vi "UHR-Fleezers Control (host) - 10.0.vi"() -> ()   [LabVIEW 2009] (continued)
  # "Harvard Pump\n(sample channel for flow exp)"
  # "Chemyx Pump 2"
  # "Units: \n1 = ml/m\n2 = ml/h\n3 = ul/m\n4 = ul/h"
  # "Rate param is ul/h\nVolume param is ul"
  # "X"
  # "Y"
  # "Oscillate Set 1 freq. (debugging)"
  # "BD 1"
  # "BD 2"
  # "AOD Raster Scan"
  # "Approx. trap separations"
  # "X"
  # "Y"
  # "APD Gates"
  # "APD 2"
  # "APD 1"
  # "X"
  # "2D"
  # "Y"
  # "1D"
  # "Green Laser Interlacing"
  # "Green FB Measurement"
  # "Digital Gate"
  # "Current Analog Control"
  # "Total AI Rates (NOT rates/trap)"
  # "(Samples/trap x Trap Sets)"
  # "(Samples/channel x\n8 if averaging (8 channels)\n4 if no averaging)"
  # "Trap 1"
  # "Trap 2"
  # "Flour./Trap 3"
  # "External Video Window"
  # "MCL Position Debugging"
  # "Temporary Control Storage\n(these used to be somewhere else, still want to keep them)"
  # "Y"
  # "X"
  # "Trap Position Difference Limits"
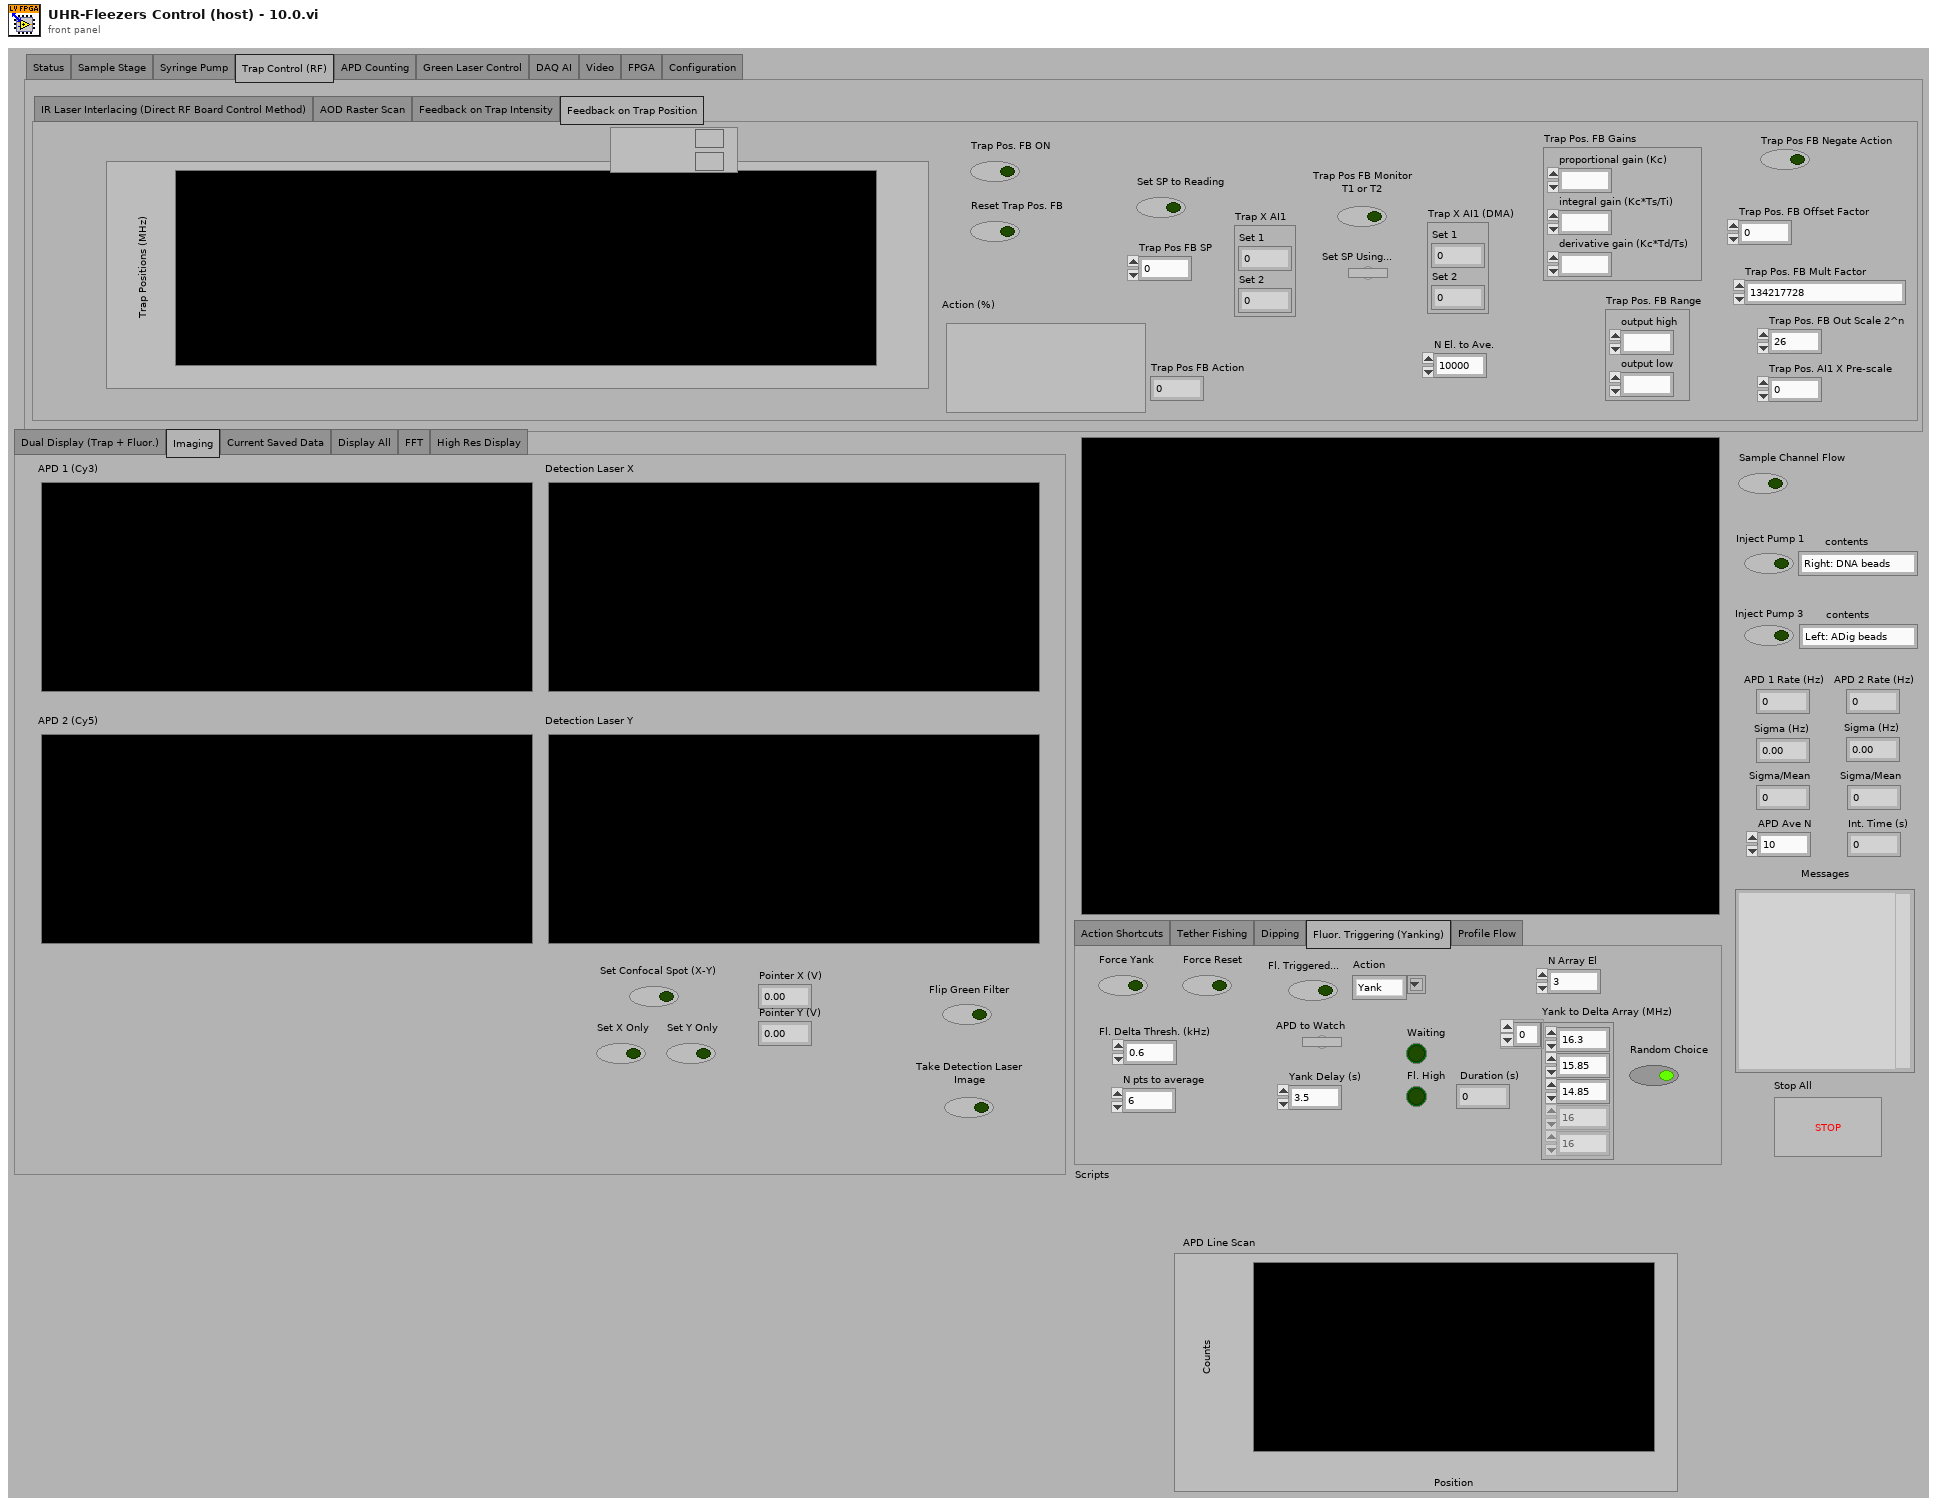
[diagram p1: front panel]
types:
  T1 = enum32{"Action Shortcuts", "Tether Fishing", "Dipping", "Fluor. Triggering (Yanking)", "Profile Flow"}
  T2 = typedef "IMAQ Image.ctl" = refnum<image>
  T3 = enum32{"Dual Display (Trap + Fluor.)", "Imaging", "Current Saved Data", "Display All", "FFT", "High Res Display"}
  T4 = enum32{"Status", "Sample Stage", "Syringe Pump", "Trap Control (RF)", "APD Counting", "Green Laser Control", "DAQ AI", "Video", "FPGA", "Configuration"}
  T5 = cluster{"Pump 1":cluster{"Diameter (mm)":dbl, "Units":dbl, "Volume":dbl, "Rate":dbl}, "Pump 2":cluster{"Diameter (mm)":dbl, "Units":dbl, "Volume":dbl, "Rate":dbl}, "Pump 3":cluster{"Diameter (mm)":dbl, "Units":dbl, "Volume":dbl, "Rate":dbl}}
  T6 = enum32{"IR Laser Interlacing (Direct RF Board Control Method)", "AOD Raster Scan", "Feedback on Trap Intensity", "Feedback on Trap Position"}
  T7 = typedef "LVPoint32TypeDef.ctl" = cluster{"Horizontal":i32, "Vertical":i32}
  T8 = cluster{"Scan Range AOD (nm) 2":dbl, "Step Size AOD (nm) 2":dbl, "Scan Speed AOD (nm/s) 2":dbl, "Number of scans (AOD) 2":u16, "Label":string}[]
  T9 = cluster{"Set 1":cluster{"proportional gain (Kc)":i16, "integral gain (Kc*Ts/Ti)":i16, "derivative gain (Kc*Td/Ts)":i16}, "Set 2":cluster{"proportional gain (Kc)":i16, "integral gain (Kc*Ts/Ti)":i16, "derivative gain (Kc*Td/Ts)":i16}}
  T10 = cluster{"Set 1":fxp<+/-,16,1>, "Set 2":fxp<+/-,16,1>}
  T11 = cluster{"proportional gain (Kc)":fxp<+/-,16,8>, "integral gain (Kc*Ts/Ti)":fxp<+/-,16,8>, "derivative gain (Kc*Td/Ts)":fxp<+/-,16,8>}
  T12 = cluster{"output high":fxp<+/-,16,1>, "output low":fxp<+/-,16,1>}
  T13 = cluster{"proportional gain (Kc)":i16, "integral gain (Kc*Ts/Ti)":i16, "derivative gain (Kc*Td/Ts)":i16}
  T14 = cluster{"Set 1":bool, "Set 2":bool, "Set 3":bool}
  T15 = typedef "LVMinMaxIncTypeDef.ctl" = cluster{"Minimum":dbl, "Maximum":dbl, "Increment":dbl}
  T16 = typedef "Image Type" = u32
  T17 = typedef "nirio_resource_hc.ctl" = tag
  T18 = typedef "niFpgaNodeNameForErrorReporting.ctl" = enum16{"Open FPGA VI Reference", "Read/Write Control", "Invoke Method: Abort", "Invoke Method: Acknowledge IRQ", "Invoke Method: Download", "Invoke Method: FIFO.Configure", "Invoke Method: FIFO.Read", "Invoke Method: FIFO.Start", "Invoke Method: FIFO.Stop", "Invoke Method: FIFO.Write", "Invoke Method: Reset", "Invoke Method: Run", "Invoke Method: Wait on IRQ", "Close FPGA VI Reference"}
  T19 = typedef "niLvFpgaWhatHappensToTopLevelVI.ctl" = enum16{"top level VI scripted behind XNode", "top level VI inlined behind XNode"}
  T20 = typedef "openfpgaref.8.6.ctl" = refnum<k20>
  T21 = cluster{"New Image":T2, "New Image":T2, "New Image":T2, "New Image":T2}
  T22 = typedef "XDNodeRunTimeDep.lvlib/timing_clust.ctl" = cluster{"Expected End [f-1]":u64, "Actual End [f-1]":u64, "Finished Late? [f-1]":bool, "Expected End [i-1]":u64, "Actual End [i-1]":u64, "Finished Late? [i-1]":bool, "Expected Start [i]":u64, "Actual Start [i]":u64, "Expected Start [f]":u64, "Actual Start [f]":u64, "Source Name":string, "Structure Name":string, "Period":i64, "Deadline":i64, "Offset":i64, "Start":i64, "Priority":i32, "Timeout":i32, "Mode":T23, "Wakeup Reason":T24, "Error":errorcluster, "Source Type":string, "Secondary Source Type":string, "Global End Time":u64, "Global Start Time":u64, "Frame Duration":u64, "Iteration Duration":u64, "Assigned CPU":i32, "I/O Scan Engine Mode":u32}
  T23 = typedef "XDNodeRunTimeDep.lvlib/nitl_modes.ctl" = enum32{"No Change", "Process missed periods, maintain original phase", "Discard missed periods, maintain original phase", "Process missed periods, ignore original phase", "Discard missed periods, ignore original phase"}
  T24 = typedef "XDNodeRunTimeDep.lvlib/wakeup.ctl" = enum32{"Normal", "Aborted", "Asynchronous wakeup", "Timing source error", "Timed loop error", "Timeout"}
  T25 = enum32{"Normal Display", "Dual Display (APD)", "FFT", "High Res Display"}
  T26 = cluster{"Origin Pixel":cluster{"X":sgl, "Y":sgl}, "Angle Relative to Horizontal (deg)":sgl, "Axis Reference":u32}
  T27 = typedef "Simple Grid Descriptor" = cluster{"X Step":sgl, "Y Step":sgl, "Unit":T28}
  T28 = typedef "Image Unit" = enum32{"Undefined", "Angström", "Micrometer", "Millimeter", "Centimeter", "Meter", "Kilometer", "Microinch", "Inch", "Feet", "Nautical miles", "Standard miles", "Steps"}
  T29 = cluster{"averaging mode":u16, "weighting mode":u16, "number of averages":u32}
  T30 = cluster{"dB On (F)":bool, "unwrap phase (F)":bool, "convert to degree (F)":bool}
  T31 = cluster{"Green FB Ch 0":i16, "Green FB Ch 1":i16, "Green FB Ch 2":i16}
  T32 = enum16{"open", "replace", "create", "open or create", "replace or create", "replace or create with confirmation"}
  T33 = enum16{"big-endian, network order", "native, host order", "little-endian"}
  T34 = cluster{string, string, string, string, string, string, string, string}
  T35 = cluster{string, string, string, string, string, string, string, string, string, string, string, string}
  T36 = cluster{string, string, string, string, string, string, string, string, string, string, string, string, string}
  T37 = cluster{string, string, string, string, string, string, string, string, string, string, string, string, string, string}
  T38 = cluster{"f0":dbl, "df":dbl, "magnitude":dbl[]}[][]
  T39 = cluster{"Green FB Ch 0":dbl, "Green FB Ch 1":dbl, "Green FB Ch 2":dbl}
  T40 = enum32{"setting", "request", "request control", "info", "statistics", "system settings", "I/O sub system", "HRT control", "camera descriptions", "device specific data", "event sub system settings", "event sub system results", "image memory manager"}
  T41 = typedef "AviRefnum.ctl" = refnum<k1>
  T42 = typedef "imagedata.ctl" = cluster{"image type":i32, "image depth":i32, "image":u8[], "mask":u8[], "colors":u32[], "Rectangle":cluster{"left":i16, "top":i16, "right":i16, "bottom":i16}}
  T43 = cluster{"Scan Range AOD (nm) 2":dbl, "Step Size AOD (nm) 2":dbl, "Scan Speed AOD (nm/s) 2":dbl, "Number of scans (AOD) 2":u16, "Label":string}
  T44 = cluster{"[0]":dbl, "[1]":dbl, "[2]":dbl, "[3]":dbl, "[4]":dbl, "[5]":dbl}
  T45 = cluster{"Diameter (mm)":dbl, "Units":dbl, "Volume":dbl, "Rate":dbl}
  T46 = cluster{"Left":i32, "Top":i32, "Width":u32, "Height":u32}
  T47 = cluster{cluster{"Left":i32, "Top":i32, "Width":u32, "Height":u32}}[]
diagram:
  w25 = u16 20 items=["1.0"=10, "1.5"=15, "2.0"=20] ("stop bits (10: 1 bit)")
  w32 = T16 2 items=["Grayscale (U8)", "Grayscale (I16)", "Grayscale (SGL)", "Complex (CSG)", "RGB (U32)", "HSL (U32)", "RGB (U64)", "Grayscale (U16)"] ("Image Type")
  w102 = cluster{"output high":i16, "output low":i16} {"output high"=3000, "output low"=0} ("FB output range 1")
  w10 = TRUE ("AI to FIFO")
  w190 = 10.0 ("y")
  w189 = 32767.0 ("y")
  w205 = 6.0  # clock mult.
  w206 = 49152000.0  # TCXO frequ.
  w9 = FALSE ("AI to FIFO")
  # "Trap data still won't flow until AI to FIFO\nis ON.  But turn trap on first to make sure they\nboth start at the same time."
  n1 = Build Array("DIO count 1 (ticks)", "DIO count 2 (ticks)", "DIO count 3 (ticks)") -> (w89:u32[])
  n2 = Multiply(x="APD Integration Time (s)", y=40000000.0) -> (x*y=w113:dbl)
  n3 = Reciprocal(x="APD Integration Time (s)") -> (1/x=w110:dbl)
  n4 = local write "APD Acq Rate (Hz)"(w110) -> ()
  n5 = local read "AO1"() -> (w184:dbl)
  n6 = local read "AO2"() -> (w183:dbl)
  n7 = To Unsigned Long Integer(number=w113) -> (unsigned 32bit integer=w112:u32)
  "APD Int. Count" <- w112
  n8 = local read "Scan Increment (MHz)"() -> (w201:dbl)
  n9 = local read "Continuous MCL Scanning"() -> (w171:bool)
  n10 = local read "Fast Scan Dir"() -> (w170:bool)
  n11 = Multiply(x=w184, y=w189) -> (x*y=w186:dbl)
  n12 = local read "Number of scans (MCL)"() -> (w172:u64)
  n13 = Multiply(x=w183, y=w189) -> (x*y=w188:dbl)
  n14 = Divide(x=w186, y=w190) -> (x/y=w185:dbl)
  n15 = Divide(x=w188, y=w190) -> (x/y=w187:dbl)
  n16 = To Word Integer(number=w185) -> (16bit integer=w182:i16)
  n17 = To Word Integer(number=w187) -> (16bit integer=w181:i16)
  n18 = Not(x=w170) -> (.not. x?=w165:bool)
  n19 = local read "Cycles/step (MCL)"() -> (w173:u64)
  n20 = Multiply(x=w201, y=1000.0) -> (x*y=w208:dbl)
  n21 = local read "Scan steps (MCL)"() -> (w174:u64)
  n22 = local read "Desired Scan Incr (V)"() -> (w176:dbl)
  n23 = Scale By Power Of 2(n=48, x=w208) -> (x*2^n=w209:dbl)
  n24 = Multiply(x=w206, y=w205) -> (x*y=w204:dbl)
  n25 = Divide(x=w209, y=w204) -> (x/y=w203:dbl)
  n26 = local read "Setpoints (V)"() -> (w224:cluster{"Set 1":dbl, "Set 2":dbl})
  n27 = property on="AI Count (ticks)" class="DigNum (strict)"("Val(Sgnl)"="AI Count (ticks)") -> ()  [unwired: 2 in, 2 out]
  n28 = local read "Number Interlace Sets"() -> (w82:u8)
  n29 = Split 1D Array(array=w89, index=w82) -> (first subarray=w91:u32[])  [unwired: 1 out]
  n30 = Add Array Elements(numeric array=w91) -> (sum=w90:u32)
  n31 = local read "# Samples/channel"() -> (w193:u32)
  n32 = To Quad Integer(1:w203) -> (0:w200:i64)
  n33 = local read "Sets to FIFO (Traps)"() -> (w231:T14)
  n34 = local read "Number of F/B Scans (AOD)"() -> (w194:u16)
  n35 = local read "Not-Interlacing Set"() -> (w81:enum32{"Set 1", "Set 2", "Set 3"})
  n36 = To Unsigned Byte Integer(number=w81) -> (unsigned 8bit integer=w87:u8)
  n37 = Index Array(array=w89, index=w87) -> (element=w88:u32)
  n38 = Divide(x=40000000.0, y="AI Count (ticks)") -> (x/y=w161:dbl)
  n39 = Multiply(x=w176, y=32767.0) -> (x*y=w178:dbl)
  n40 = local read "Feedback On/Off"() -> (w227:cluster{"Set 1":bool, "Set 2":bool})
  n41 = local read "PID Gains"() -> (w219:T9)
  n42 = local read "Scan steps (AOD)"() -> (w199:u64)
  n43 = local read "All FB On/Off"() -> (w228:bool)
  n44 = local read "Cycles/step (AOD)"() -> (w198:u64)
  n45 = local write "AI rate (Hz)"(w161) -> ()
  n46 = Divide(x=w178, y=10.0) -> (x/y=w177:dbl)
  n47 = Multiply(x=w199, y=w198) -> (x*y=w197:u64)
  n48 = Multiply(x=3276.7, y=w224) -> (x*y=w223:cluster{"Set 1":dbl, "Set 2":dbl})
  n49 = To Word Integer(number=w177) -> (16bit integer=w175:i16)
  n50 = Multiply(x=w197, y=u64 2) -> (x*y=w195:u64)
  n51 = Divide(x=w161, y="FPGA Ave.") -> (x/y=w162:dbl)
  n52 = To Word Integer(number=w223) -> (16bit integer=w222:cluster{"Set 1":i16, "Set 2":i16})
  n53 = xnode "Open FPGA VI Reference"("resource name"=T17 "750kHzDAQ") -> ("FPGA VI Reference Out"=w216:refnum<k20>, "error out"=w215:errorcluster)  [unwired: 1 in]
  n54 = Unbundle By Name(w219) -> ("Set 1"=w218:T13, "Set 2"=w217:T13)
  n55 = Multiply(x=w195, y=w194) -> (x*y=w192:u64)
  n56 = Divide(x=w192, y=w193) -> (x/y=w191:dbl)
  n57 = local write "Ave. Rate (Hz)"(w162) -> ()
  n58 = Unbundle By Name(w222) -> ("Set 1"=w221:i16, "Set 2"=w220:i16)
  n59 = local read "2D or 1D Scan"() -> (w105:bool)
  n60 = local write "Data points/scans"(w192) -> ()
  n61 = And(x=w227, y=w228) -> (x .and. y?=w226:cluster{"Set 1":bool, "Set 2":bool})
  n62 = local read "Scan BD"() -> (w210:bool)
  n63 = Reciprocal(x=w162) -> (1/x=w163:dbl)
  n64 = local write "Data points/scan (f/b)"(w195) -> ()
  n65 = local read "N Acq Sets (Traps + Fl.)"() -> (w154:i16)
  n66 = local write "N sets should be saved"(w191) -> ()
  n67 = Unbundle By Name(w226) -> ("Set 1"=w230:bool, "Set 2"=w229:bool)
  n68 = xnode "Invoke Method"("FPGA VI Reference In"=w216, "error in"=w215) -> ("FPGA VI Reference Out"=w101:refnum<k20>, "error out"=w128:errorcluster)
  n69 = local read "Interlace"() -> (w83:bool)
  n70 = Select(t=w90, s=w83, f=w88) -> (s? t:f=w80:u32)
  n71 = local write "Update Count (MCL)"(w80) -> ()
  n72 = local write "Total Counts (ticks)"(w80) -> ()
  n73 = local write "Ave. Period (s)"(w163) -> ()
  n74 = property on="2D or 1D Scan" class="Bool (strict)"("Val(Sgnl)"=w105) -> ()  [unwired: 2 in, 2 out]
  n75 = xnode "Read/Write Control"("FPGA VI Reference In"=w100, "error in"=w128, "ai count"="AI Count (ticks)", "AI Averages"="FPGA Ave.", "DMA buffer timeout"=0, "AI to FIFO"=w9, "Trap Pos to FIFO"=w9, "Interlace ON/OFF"=w83, "Number Interlace Cycles"=w82, "AI1 Sets to FIFO"=w231, "FB On/Off Set 1"=w230, "FB On/Off Set 2"=w229, "Interlace Off Parameters"=w81, "FB Setpoint Set 1"=w221, "FB Setpoint Set 2"=w220, "FB Gains Set 1"=w218, "FB Gains Set 2"=w217, "FB output range 1"=w102, "FB output range 2"=w102, "Cycles per step"=w198, "Scan BD"=w210, "Number of scans"=w194, "Scan steps"=w199, "Scan freq.  increment"=w200, "AO1"=w182, "AO2"=w181, "Scan freq.  increment (MCL)"=w175, "Scan steps (MCL)"=w174, "Cycles per step (MCL)"=w173, "Number of scans (MCL)"=w172, "MCL count"=w80, "Cont. Scan (MCL)"=w171, "MCL Scan Axis"=w165, "1D or 2D Scan?"=w105, "N of AI1 Int Acq Sets"=w154, "Freq or Amp switch first"="Freq or Amp switch first", "Freq switch delay"="Freq switch delay", "Amp switch delay"="Amp switch delay", "Swap F1 and F2"="Swap F1 and F2", "APD Acq Rate Count"=w112, "APD to FIFO"=FALSE, "APD Gate Operating Mode"="APD Gate", "APD Gate ON Count"="APD Gate ON Count", "APD Gate OFF Count"="APD Gate OFF Count", "Invert APD Gate"="Invert APD Gate", "DIO count 1 (ticks)"="DIO count 1 (ticks)", "DIO count 2 (ticks)"="DIO count 2 (ticks)", "DIO count 3 (ticks)"="DIO count 3 (ticks)", "APD 1 AO scale factor"="APD 1 AO Mult.", "APD 2 AO scale factor"="APD 2 AO Mult.", "APD 1 AO offset"="APD 1 AO offset", "APD 2 AO offset"="APD 2 AO offset") -> ("FPGA VI Reference Out"=w75:refnum<k20>, "error out"=w77:errorcluster)
  n76 = local read "Green Laser ON/Interlacing"() -> (w78:bool)
  n77 = local read "Green laser mode"() -> (w79:enum32{"Laser ON", "Laser OFF", "Interlace"})
  n78 = local read "GI Frequency, OFF count"() -> (w71:u32)
  n79 = local read "GI Frequency, ON count"() -> (w70:u32)
  n80 = Multiply(x="Current When FB OFF (%)", y=655.35) -> (x*y=w61:dbl)
  n81 = local read "Green FB Count"() -> (w69:u32)
  n82 = Multiply(x="Green FB Setpoint (mV)", y=3.2767) -> (x*y=w58:dbl)
  n83 = To Unsigned Word Integer(number=w61) -> (unsigned 16bit integer=w59:u16)
  n84 = local read "Invert GI"() -> (w73:bool)
  n85 = To Word Integer(number=w58) -> (16bit integer=w56:i16)
  n86 = case shown="False" w78 {
    tunnel: w79 -> [_ w257]
    tunnel: [enum32{"Laser ON", "Laser OFF", "Interlace"}."Laser OFF" ("Green laser mode") w257] -> w72
    frame #0 {
    }
    frame #1 {
    }
  }
  n87 = local read "Trap Pos. AI1 X Pre-scale"() -> (w1:u16)
  n88 = local read "Trap Pos FB Monitor\nT1 or T2"() -> (w8:bool)
  n89 = local read "Trap Pos FB Negate Action"() -> (w7:bool)
  n90 = local read "Trap Pos. FB Offset Factor"() -> (w6:i64)
  n91 = local read "Trap Pos. FB Mult Factor"() -> (w5:i64)
  n92 = local read "Trap Pos. FB Gains"() -> (w3:T11)
  n93 = local read "Trap Pos. FB Range"() -> (w4:T12)
  n94 = xnode "Read/Write Control"("FPGA VI Reference In"=w75, "error in"=w77, "Green interlace ON count 2"=w70, "Green interlace OFF count 2"=w71, "Invert GI 2"=w73, "Operating Mode 2"=w72, "Green FB Gains"="Green FB Gains", "Green FB Setpoint"=w56, "Green FB On/Off"="Green FB On/Off", "Current Out"=w59, "Green int current ON count adj"="Green int current ON count adj", "Green FB Count"=w69, "Operating Mode"=w72, "Green interlace OFF count"=w71, "Green interlace ON count"=w70, "Invert GI"=w73, "APD2 Trigger on Edge?"="APD2 Trigger on Edge?", "APD1 Trigger on Edge?"="APD1 Trigger on Edge?", "Trap Pos FB Monitor T1 or T2"=w8, "Trap Pos FB Negate Action"=w7, "Trap Pos. FB Offset Factor"=w6, "Trap Pos. FB Mult Factor"=w5, "Trap Pos. FB Range"=w4, "Trap Pos. FB Gains"=w3, "Force feedback"=FALSE, "AI1 X Scale"=w1) -> ("FPGA VI Reference Out"=w74:refnum<k20>, "error out"=w76:errorcluster)  [unwired: 1 in]
  n95 = xnode "Invoke Method"("FPGA VI Reference In"=w74, "error in"=w76, "Depth"="Trap AI FIFO Depth") -> ("FPGA VI Reference Out"=w21:refnum<k20>, "error out"=w20:errorcluster)
  n96 = xnode "Invoke Method"("FPGA VI Reference In"=w21, "error in"=w20, "Depth"="Trap Position FIFO Depth") -> ("FPGA VI Reference Out"=w18:refnum<k20>, "error out"=w17:errorcluster)
  n97 = xnode "Invoke Method"("FPGA VI Reference In"=w18, "error in"=w17) -> ("FPGA VI Reference Out"=w16:refnum<k20>, "error out"=w15:errorcluster)
  n98 = flat-sequence {
    tunnel: w101 -> [w262]
    tunnel: [w262] -> w100
    tunnel: [w261] -> w99
    tunnel: [w260] -> w98
    tunnel: [w258] -> w96
    tunnel: [w259] -> w97
    frame #0 {
      w259 = T15 {"Minimum"=0.0, "Maximum"=40.0, "Increment"=1.0} ("Min Max Inc")
      w258 = T15 {"Minimum"=0.0, "Maximum"=50.0, "Increment"=1.0} ("Data Entry Limits")
      w261 = T15 {"Minimum"=60.0, "Maximum"=90.0, "Increment"=1.0} ("Min Max Inc")
      w260 = T15 {"Minimum"=0.0, "Maximum"=50.0, "Increment"=1.0} ("Data Entry Limits")
      n99 = property on="BD 2 Frequency 1 (MHz)" class="DigNum (strict)"("Data Range"=w259) -> ()  [unwired: 2 in, 2 out]
      n100 = property on="BD 2 Frequency 3 (MHz)" class="DigNum (strict)"("Data Range"=w259) -> ()  [unwired: 2 in, 2 out]
      n101 = property on="BD 2 Frequency 2 (MHz)" class="DigNum (strict)"("Data Range"=w259) -> ()  [unwired: 2 in, 2 out]
      n102 = property on="BD 1 Frequency 1 (MHz)" class="DigNum (strict)"("Data Range"=w261) -> ()  [unwired: 2 in, 2 out]
      n103 = property on="BD 1 Frequency 2 (MHz)" class="DigNum (strict)"("Data Range"=w261) -> ()  [unwired: 2 in, 2 out]
      n104 = property on="BD 1 Frequency 3 (MHz)" class="DigNum (strict)"("Data Range"=w261) -> ()  [unwired: 2 in, 2 out]
      n105 = property on="BD 2 Amplitude 1 (%)" class="DigNum (strict)"("Data Range"=w258) -> ()  [unwired: 2 in, 2 out]
      n106 = property on="BD 2 Amplitude 2 (%)" class="DigNum (strict)"("Data Range"=w258) -> ()  [unwired: 2 in, 2 out]
      n107 = property on="BD 2 Amplitude 3 (%)" class="DigNum (strict)"("Data Range"=w258) -> ()  [unwired: 2 in, 2 out]
      n108 = property on="BD 1 Amplitude 3 (%)" class="DigNum (strict)"("Data Range"=w260) -> ()  [unwired: 2 in, 2 out]
      n109 = property on="BD 1 Amplitude 2 (%)" class="DigNum (strict)"("Data Range"=w260) -> ()  [unwired: 2 in, 2 out]
      n110 = property on="BD 1 Amplitude 1 (%)" class="DigNum (strict)"("Data Range"=w260) -> ()  [unwired: 2 in, 2 out]
      "X RF Frequency Limits (MHz)" <- w261
      "X RF Amplitude Limits (%)" <- w260
      "Y RF Amplitude Limits (%)" <- w258
      "Y RF Frequency Limits (MHz)" <- w259
    }
  }
  n111 = xnode "Invoke Method"("FPGA VI Reference In"=w16, "error in"=w15) -> ("FPGA VI Reference Out"=w127:refnum<k20>, "error out"=w126:errorcluster)
  n112 = xnode "Invoke Method"("FPGA VI Reference In"=w127, "error in"=w126) -> ("FPGA VI Reference Out"=w125:refnum<k20>, "error out"=w124:errorcluster)  [unwired: 1 out]
  n113 = flat-sequence "Initial FPGA Loop Relative Phase Adjustment" {
    tunnel: "Initial Phase Adjustment (AI1)" -> [w273]
    tunnel: "Initial Phase Adjustment (GI)" -> [w272]
    tunnel: w125 -> [w271]
    tunnel: w124 -> [w270]
    tunnel: "Initial Phase Adj. (MCL)" -> [w269]
    tunnel: [w274] -> w136
    tunnel: [w268] -> w132
    tunnel: "Initial Phase Adjustment (APD Acq)" -> [w267]
    tunnel: "Initial Phase Adjustment (APD 1 Gate)" -> [w266]
    tunnel: "Initial Phase Adjustment (Green FB)" -> [w265]
    tunnel: "Initial Phase Adjustment (GI) 2" -> [w264]
    tunnel: "Initial Phase Adjustment (APD 2 Gate)" -> [w263]
    tunnel: w136 -> [w445]
    tunnel: [w446] -> w133
    tunnel: w132 -> [w446]
    tunnel: [w445] -> w131
    tunnel: w133 -> [w449]
    tunnel: w131 -> [w448]
    tunnel: [w451] -> w130
    tunnel: [w450] -> w129
    tunnel: [w630] -> w134
    tunnel: [w631] -> w135
    tunnel: w130 -> [w631]
    tunnel: w129 -> [w630]
    frame #0 {
      n114 = xnode "Read/Write Control"("FPGA VI Reference In"=w271, "error in"=w270, "Phase count adjustment"=w273, "Phase count adjustment (GI)"=w272, "Phase count adjustment (MCL)"=w269, "Phase Count Adjustment (APD Acq)"=w267, "Phase count adjustment (APD 1 Gate)"=w266, "Phase count adjustment (APD 2 Gate)"=w263, "Phase count adjustment (Green FB)"=w265, "Phase count adjustment (GI) 2"=w264) -> ("FPGA VI Reference Out"=w268:refnum<k20>, "error out"=w274:errorcluster)
    }
    frame #1 {
      n115 = Wait (ms)(milliseconds to wait=u32 1000) -> ()  [unwired: 1 out]
    }
    frame #2 {
      w447 = TRUE
      n116 = xnode "Read/Write Control"("FPGA VI Reference In"=w449, "error in"=w448, "+ phase"=w447, "+ phase (GI)"=w447, "+ phase (MCL)"=w447, "+ phase (APD Acq)"=w447, "+ phase (APD 1 Gate)"=w447, "+ phase (APD 2 Gate)"=w447, "+ phase (Green FB)"=w447, "+ phase (GI) 2"=w447) -> ("FPGA VI Reference Out"=w450:refnum<k20>, "error out"=w451:errorcluster)
    }
    frame #3 {
      n117 = Wait (ms)(milliseconds to wait=u32 1000) -> ()  [unwired: 1 out]
    }
  }
  n118 = local read "Phase adj. (Green FB)"() -> (w92:i16)
  n119 = local read "Phase adj. (GI) 2"() -> (w62:i16)
  n120 = local read "Phase adjust (MCL)"() -> (w166:i16)
  n121 = local read "Phase adj. (AI1)"() -> (w168:i16)
  n122 = local read "Phase adj. (GI)"() -> (w167:i16)
  n123 = xnode "Read/Write Control"("FPGA VI Reference In"=w134, "error in"=w135, "Phase count adjustment"=w168, "Phase count adjustment (GI)"=w167, "Phase count adjustment (MCL)"=w166, "Phase Count Adjustment (APD Acq)"="Phase Adj. (APD Acq)", "Phase count adjustment (APD 1 Gate)"="Phase Adj. (APD 1 Gate)", "Phase count adjustment (APD 2 Gate)"="Phase Adj. (APD 2 Gate)", "Phase count adjustment (Green FB)"=w92, "Phase count adjustment (GI) 2"=w62) -> ("FPGA VI Reference Out"=w48:refnum<k20>, "error out"=w143:errorcluster)
  n124 = call "Initialize RF boards - interlace 3.vi"("error in"=w143, "FPGA VI Reference In"=w48) -> ("error out"=w141:errorcluster, "FPGA VI Reference Out"=w142:T20)
  n125 = call "set RF board frequency - interlace.vi"("Board 2 Frequency Limits"=w97, "Board 1 Frequency Limits"=w99, "error in"=w141, "FPGA VI Reference In"=w142, "Board 2 Frequency 3 (MHz)"="BD 2 Frequency 3 (MHz)", "Board 1 Frequency 3 (MHz)"="BD 1 Frequency 3 (MHz)", "Board 2 Frequency 2 (MHz)"="BD 2 Frequency 2 (MHz)", "Board 2 Frequency 1 (MHz)"="BD 2 Frequency 1 (MHz)", "Board 1 Frequency 2 (MHz)"="BD 1 Frequency 2 (MHz)", "Board 1 Frequency 1  (MHz)"="BD 1 Frequency 1 (MHz)") -> ("error out"=w246:errorcluster, "FPGA VI Reference Out"=w247:T20)
  n126 = call "set RF board amplitude - interlace.vi"("Board 2 Amplitude Limits"=w96, "Board 1 Amplitude Limits"=w98, "error in"=w246, "FPGA VI Reference In"=w247, "Board 2 Amplitude 3 (%)"="BD 2 Amplitude 3 (%)", "Board 1 Amplitude 3 (%)"="BD 1 Amplitude 3 (%)", "Board 2 Amplitude 2 (%)"="BD 2 Amplitude 2 (%)", "Board 2 Amplitude 1 (%)"="BD 2 Amplitude 1 (%)", "Board 1 Amplitude 2 (%)"="BD 1 Amplitude 2 (%)", "Board 1 Amplitude 1 (%)"="BD 1 Amplitude 1 (%)") -> ("error out"=w234:errorcluster, "FPGA VI Reference Out"=w235:T20)
  n127 = flat-sequence {
    tunnel: w235 -> [w640]
    tunnel: w234 -> [w639]
    tunnel: [w638] -> w239
    tunnel: [w637] -> w238
    tunnel: [w681] -> w237
    tunnel: w239 -> [w681]
    tunnel: [w680] -> w236
    tunnel: w238 -> [w680]
    tunnel: w237 -> [w689]
    tunnel: w236 -> [w688]
    tunnel: [w687] -> w14
    tunnel: [w686] -> w13
    frame #0 {
      n128 = local read "Trap 1 (ON/OFF)"() -> (w632:bool)
      n129 = xnode "Read/Write Control"("FPGA VI Reference In"=w640, "error in"=w639, "Direct RF Box  Communication"=FALSE) -> ("FPGA VI Reference Out"=w638:T20, "error out"=w637:errorcluster)
      n130 = local write "Saving..."(FALSE ("Saving Data")) -> ()
      n131 = local write "Stop All"(FALSE ("Stop All")) -> ()
      n132 = local write "Index"(1.0 ("Index")) -> ()
      n133 = property on="Trap 1 ON" class="Bool (strict)"("Value"=w632) -> ()  [unwired: 2 in, 2 out]
      "Manipulating Trap" <- FALSE ("Manipulating Trap")
    }
    frame #1 {
      n134 = local read "Trap 2 (ON/OFF)"() -> (w679:bool)
      n135 = Wait (ms)(milliseconds to wait=u32 10) -> ()  [unwired: 1 out]
      n136 = property on="Trap 2 ON" class="Bool (strict)"("Val(Sgnl)"=w679) -> ()  [unwired: 2 in, 2 out]
    }
    frame #2 {
      n137 = xnode "Read/Write Control"("FPGA VI Reference In"=w689, "error in"=w688, "FPGA Controls  RF Box"=TRUE ("Direct RF Box  Communication")) -> ("FPGA VI Reference Out"=w687:T20, "error out"=w686:errorcluster)
      n138 = call "Update messages.vi"("Message to add"="UHR-Fleezers ready.", "Old message string"="") -> ("New message string"=w685:string)
      n139 = local write "Messages"(w685) -> ()
    }
  }
  n140 = Subtract(x="BD 1 Frequency 1 (MHz)", y="BD 1 Frequency 2 (MHz)") -> (x-y=w153:dbl)
  n141 = Subtract(x="BD 2 Frequency 1 (MHz)", y="BD 2 Frequency 2 (MHz)") -> (x-y=w152:dbl)
  n142 = Square(x=w152) -> (x^2=w150:dbl)
  n143 = Square(x=w153) -> (x^2=w151:dbl)
  n144 = Add(x=w151, y=w150) -> (x+y=w149:dbl)
  n145 = Square Root(x=w149) -> (sqrt(x)=w148:dbl)
  n146 = local write "Trap Delta (MHz)"(w148) -> ()
  n147 = xnode "Read/Write Control"("FPGA VI Reference In"=w14, "error in"=w13, "Trap Pos to FIFO"=w10) -> ("FPGA VI Reference Out"=w12:T20, "error out"=w11:errorcluster)
  n148 = xnode "Read/Write Control"("FPGA VI Reference In"=w12, "error in"=w11, "AI to FIFO"=w10, "APD to FIFO"=w10) -> ("FPGA VI Reference Out"=w107:T20, "error out"=w106:errorcluster)
  n149 = call-poly "VISA Configure Serial Port"("VISA resource name"="Sample Chamber Stage Serial Port") -> ("VISA resource name out"=w43:refnum<visa-resource-name>, "error out"=w44:errorcluster)  [unwired: 5 in, 8 out]
  "Stage Control Serial Error" <- w44
  n150 = call "IMAQ Create"("Image Name"="APD 1 Image", "Image Type"=w32) -> ("New Image"=w31:T2)  [unwired: 3 in, 1 out]